vi "Modelo planta H2_V2.vi"() -> ()   [LabVIEW 2024]
uses:
  <vilib>/Platform/TimedLoop/XDataNode/timing_clust.ctl
  <vilib>/Platform/TimedLoop/XDataNode/nitl_modes.ctl
  <vilib>/Platform/TimedLoop/XDataNode/wakeup.ctl
  <vilib>/Modbus/master/Create Master Instance (TCP).vi
  <vilib>/platform/TimedLoop/XDataNode/XDataNode.xnode
  <vilib>/Modbus/master/Modbus Master.lvclass
  <vilib>/OPCUA/NI OPC UA Client.lvlib
  SALICRU_MODBUS.lvlib
  S7-1200_OPCUA.lvlib
  <vilib>/Platform/TimedLoop/XDataNode/XDNodeRunTimeDep.lvlib
  SubVIs/DB_API/DB_API.lvclass
panel:
  out "DB STATUS":bool
  out "Producció d'hidrogen":dbl(graph)
  out "Humedad":dbl format="%#.4g"
  out "Temperatura":dbl format="%#.4g"
  out "Tèrmic\nExtractors":bool
  out "Relé Seguretat":bool
  out "Sobretensions":bool
  out "Baliza verde":bool
  out "Baliza amarilla":bool
  out "Baliza roja":bool
  out "value":cluster{"message":string}
  out "ELYs_Produccio_2":dbl[](array[numeric])
  out "ELYs_Produccio_1":dbl[](array[numeric])
  in  "stop":bool
  out "Corriente S":dbl
  out "Corriente R":dbl
  out "Corriente T":dbl
  out "Salida Vr":dbl
  out "Salida Vt":dbl
  out "Salida Vs":dbl
  out "EV6":bool caption="Not initialized"
  out "EV5":bool caption="Not initialized"
  out "EV4":bool caption="Not initialized"
  out "EV3":bool caption="Idle"
  out "EV2":bool caption="Not initialized"
  out "EV1":bool caption="Stand By"
  out "x-y 4":u32
  out "x-y 3":u32
  in  "Restart INV SALICRU com":bool
  in  "Restart SAI com":bool
  in  "Tab Control":T1(tab)
  out "Prod_elec_total (kg)":dbl format="%#.2g"
  out "E2.1.2":bool caption="Not initialized"
  out "E1.1":bool caption="Maintenance mode"
  out "E2.2.2":bool caption="Not initialized"
  out "E2.3.2":bool caption="Not initialized"
  out "E1.2.2":bool caption="Maintenance mode"
  out "E1.3.2":bool caption="Idle"
  out "Prod_elec_inst (g/s)":dbl format="%#.4g"
  out "Potenica Solar (Display) 2":dbl format="%#.2f"
  out "masa total G Kg 2":dbl format="%#.3f"
  out "P alta 2":dbl format="%.1f"
  out "P baja 2":dbl format="%.1f"
  out "masa total P Kg  2":dbl format="%#.3f"
  in  "SAI":bool caption="Line"
  out "Potenica SAI (Display) 3":dbl format="%#.2f"
  out "Comunicacion SAI":bool
  out "E2.1":bool caption="Not initialized"
  out "E2.2":bool caption="Not initialized"
  out "E1.3":bool caption="Idle"
  out "E1.1,2":bool caption="Maintenance mode"
  out "E2.3":bool caption="Not initialized"
  out "E1.2":bool caption="Maintenance mode"
  out "Energia solar no utilitzada":dbl(graph)
  out "Pressió tanc baixa":dynamicdata(graph)
  out "Potenica Solar (Display)":dbl format="%#.2f"
  out "Producción FC":dbl format="%#_2g"
  out "Prod electrolizadores (display)":dbl format="%#.4g"
  out "P baja":dbl format="%.1f"
  out "masa total G Kg":dbl format="%#.0f"
  out "Potència inversor solar":dynamicdata(graph)
  out "Watimetro ARPA":dbl format="%#.1f"
  out "masa total P Kg":dbl format="%#.1f"
  out "Compresor":bool
  out "P alta":dbl format="%.1f"
  out "H2 generado Total":dbl format="%#.1f"
  out "Producción Solar toral":dbl format="%#.1f"
  out "Energía acum H2 verde":dbl format="%#.1f"
  out "H2 consumido en el lab":dbl=182.6 format="%#.1f"
  out "Energía solar diaría":dbl format="%#.1f"
  out "H2 generado dia":dbl format="%#.1f"
  out "Comunicacion Inversor SALICRU":bool
  out "Tank":dbl(slide) scale=0.0..10.0
  out "CO2":dbl
  out "H2S":dbl
  out "NO2":dbl
  out "O2":dbl
  out "O3":dbl
  out "SO2":dbl
  out "CO":dbl
  out "TVOC":dbl
  out "P tanq alta (barg)":dbl(graph)
  in  "Energía acum H2 verde inicio":dbl=527.0
  in  "Producción Solar total inicio":dbl=3421.0
  in  "H2 generado inicio":dbl=202.8
  out "g H2 consumidos por la FC":dbl
  out "g comprimidos":dbl
  in  "Caudal compresor":dbl
  out "P tanq baja (barg)":dbl(graph)
  in  "Presión ini Tanq baba":dbl=28.0
  in  "Presión ini Tanq alta":dbl=220.0
  out "Energía Solar no usada (kWh)":dbl(graph)
  out "H2 acumulado diario (g)":dbl(graph)
  out "Producción instalan (g/s)":dbl(graph)
  out "Electroli ON":dbl(graph)
  out "Potencia Consumo electroli instan. (kW)":dbl(graph)
  out "Producción diaria (g)":dbl
  out "Producción instalan (g/s)":dbl
  out "Electroli ON":dbl
  out "Potencia Solar Instanta (kW)":dbl(graph)
  # "Seguretat"
  # "EV1"
  # "EV4"
  # "ESTADO ELECTROVÁLVULAS"
  # "EV5"
  # "EV2"
  # "EV3"
  # "EV6"
  # "g"
  # "bar"
  # "bar"
  # "kg"
  # "kWh"
  # "kWh"
  # "Ambiente"
  # "Temperatura"
  # "ºC"
  # "Humedad"
  # "%"
  # "ESTADO ELY"
  # "E1.1"
  # "E2.1"
  # "E1.2"
  # "E2.2"
  # "E2.3"
  # "E1.3"
  # "Modo:"
  # "RESUMEN DE LA PRODUCCIÓN"
  # "Electrolizadores"
  # "Producción\nInstantanea:"
  # "g/s"
  # "Producción\nTotal:"
  # "kg"
  # "SAI PLANTA"
  # "Inversor solar:"
  # "Energía solar:"
  # "kW"
  # "Tanque Alta"
  # "Presión:"
  # "barg"
  # "Kg"
  # "Capacidad:"
  # "Tanque Baja"
  # "Presión:"
  # "barg"
  # "Kg"
  # "Capacidad:"
  # "SAI:"
  # "Potencia (%):"
  # "%"
  # "Hidrògen"
  # "H2 baixa pressió"
  # "H2 alta pressió"
  # "Aigua"
  # "barg"
  # "Tanc baixa pressió"
  # "Tanc alta pressió"
  # "Compressor"
  # "barg"
  # "Solar"
  # "Fuel Cell"
  # "kW"
  # "kW"
  # "kg"
  # "kg"
  # "Electrolizadors"
  # "g/s"
  # "Xarxa electrica"
  # "-"
  # "+"
  # "kW de xarxa"
  # "Producció total d'hidrogen"
  # "Producció d'hidrogen diària"
  # "g"
  # "kg"
  # "Producció total d'energia solar"
  # "Energia solar produïda diària"
  # "kWh"
  # "kWh"
  # "Energia acumulada per H2 verd"
  # "Consum de H2 Lab diari"
  # "g"
  # "kWh"
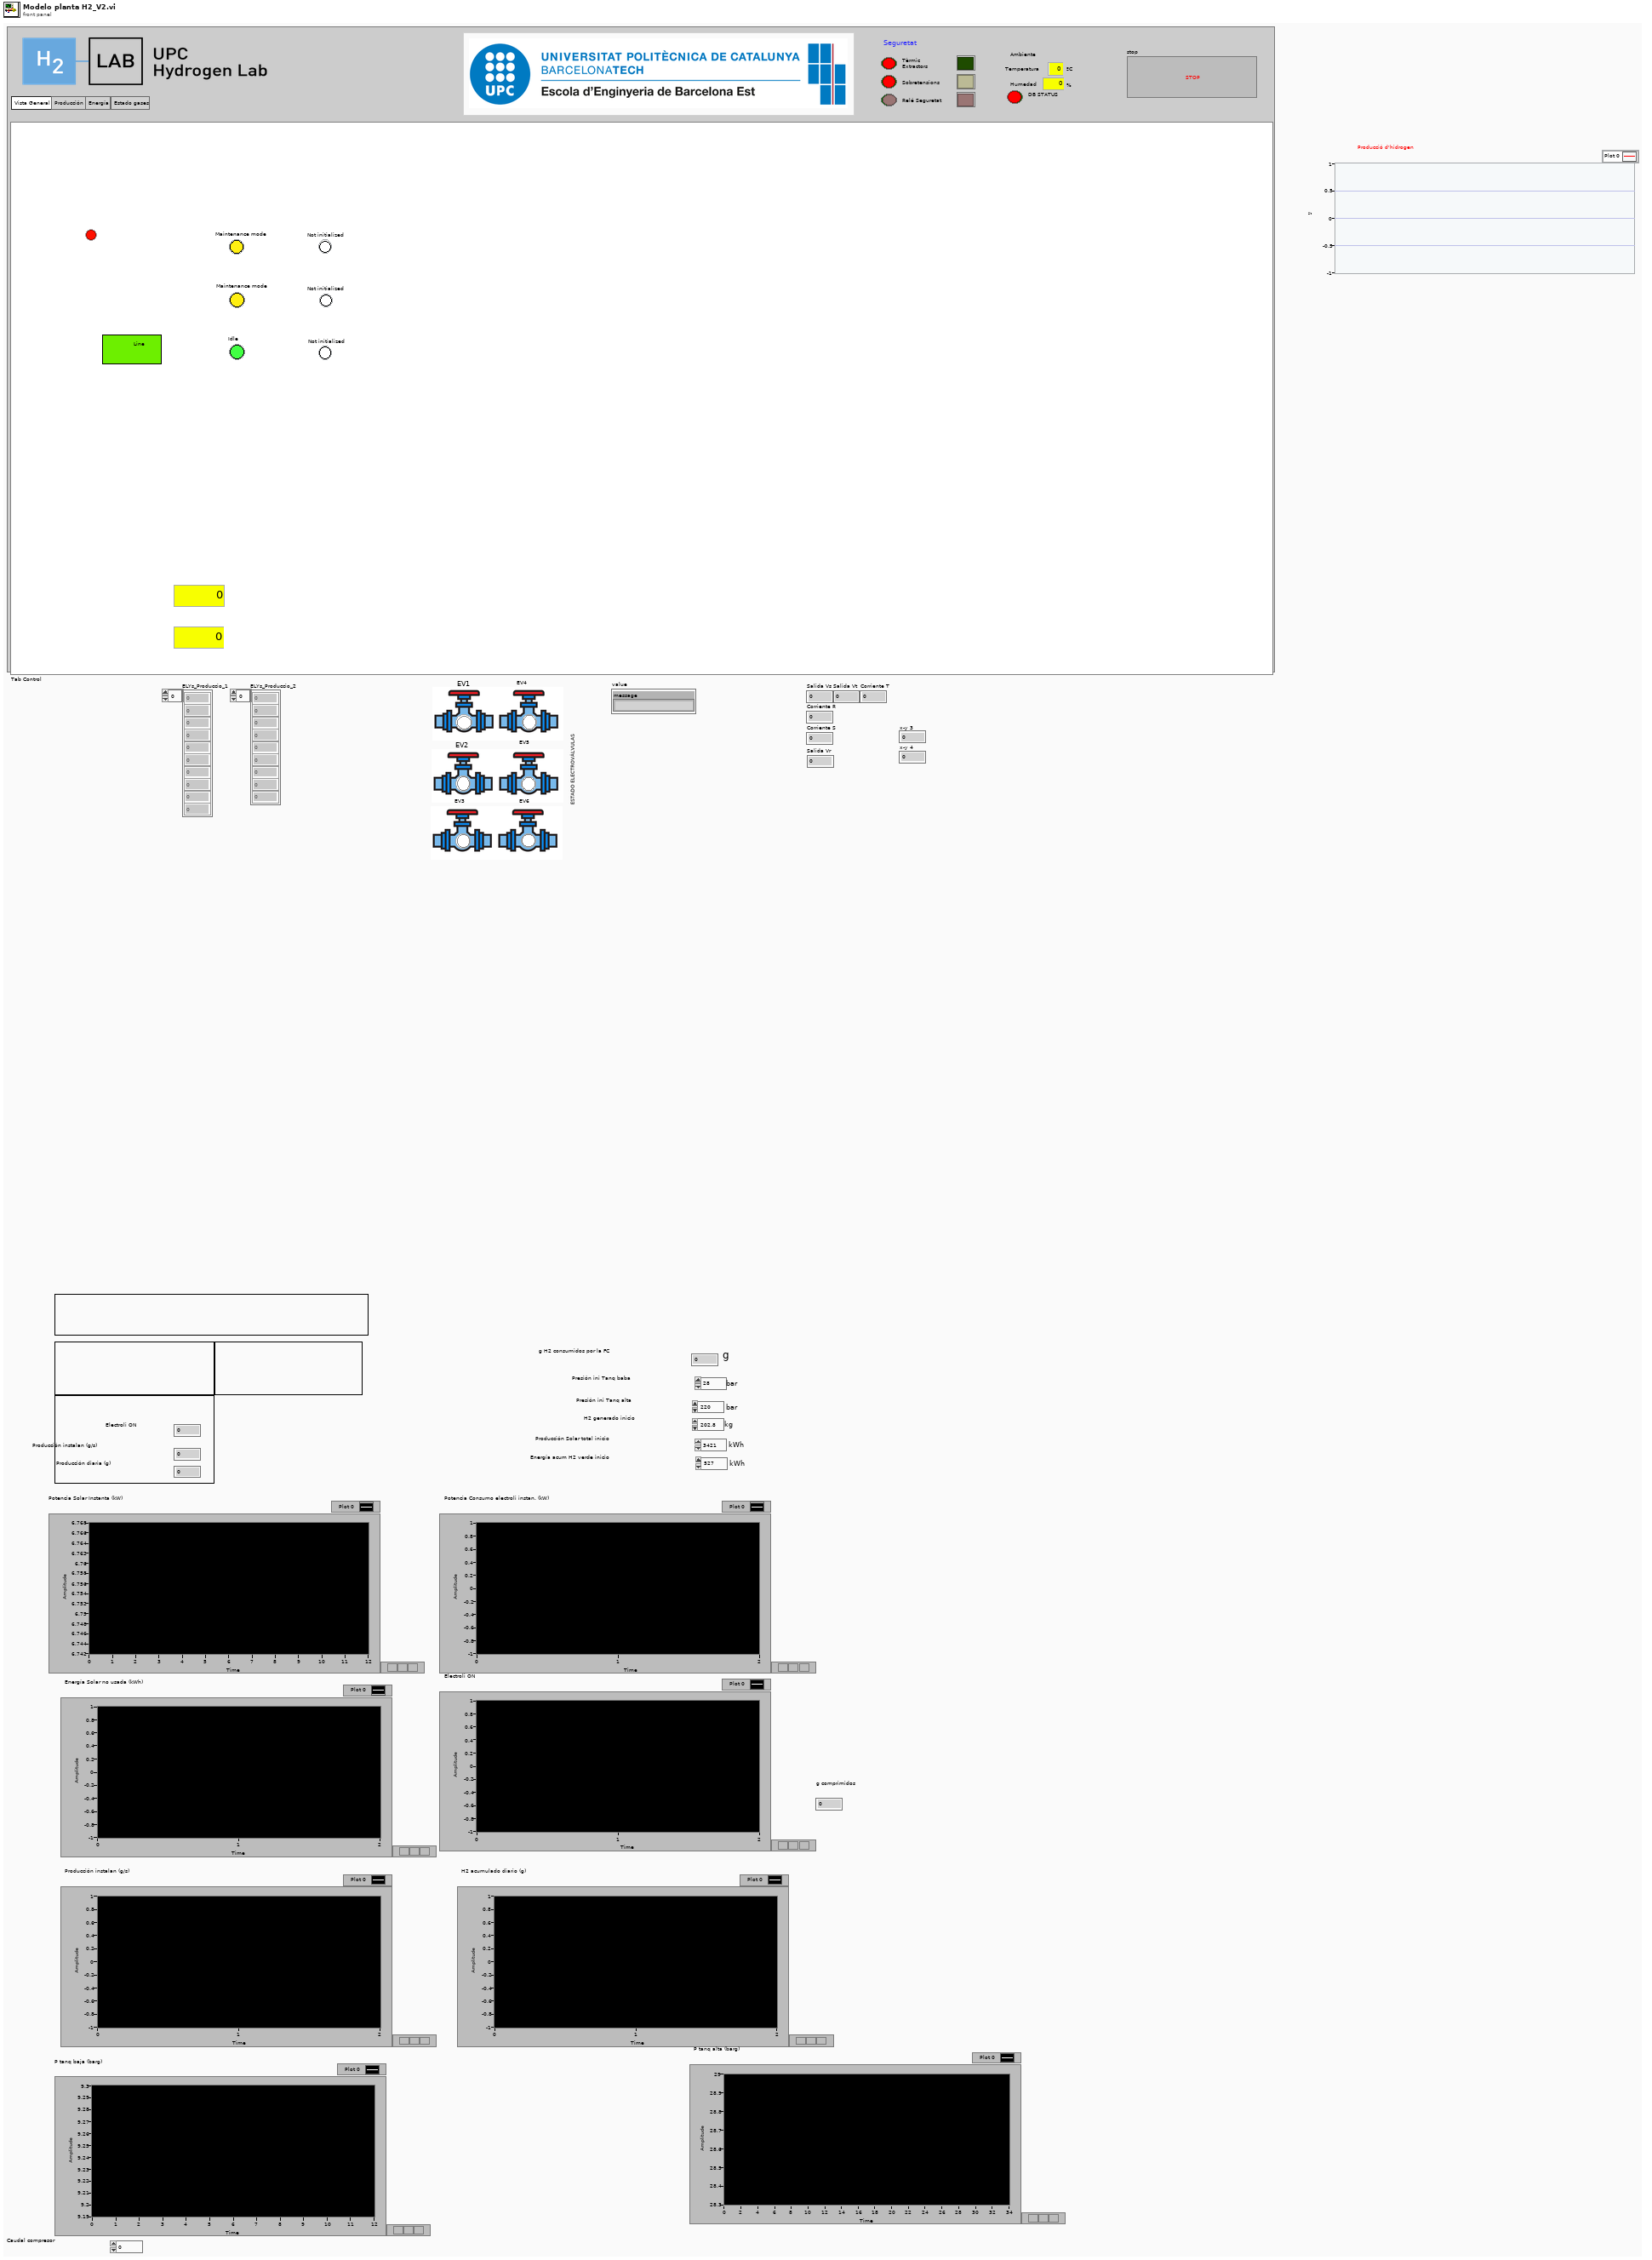
[diagram p1: front panel]
types:
  T1 = enum32{"Vista General", "Producción", "Energía", "Estado gases"}
  T2 = cluster{"message mode":enum16{"None", "Sign", "Sign and Encrypt"}, "security":enum16{"Basic256", "Basic128Rsa15"}}
  T3 = typedef "XDNodeRunTimeDep.lvlib/timing_clust.ctl" = cluster{"Expected End [f-1]":u64, "Actual End [f-1]":u64, "Finished Late? [f-1]":bool, "Expected End [i-1]":u64, "Actual End [i-1]":u64, "Finished Late? [i-1]":bool, "Expected Start [i]":u64, "Actual Start [i]":u64, "Expected Start [f]":u64, "Actual Start [f]":u64, "Source Name":string, "Structure Name":string, "Period":i64, "Deadline":i64, "Offset":i64, "Start":i64, "Priority":i32, "Timeout":i32, "Mode":T4, "Wakeup Reason":T5, "Error":errorcluster, "Source Type":string, "Secondary Source Type":string, "Global End Time":u64, "Global Start Time":u64, "Frame Duration":u64, "Iteration Duration":u64, "Assigned CPU":i32, "I/O Scan Engine Mode":u32}
  T4 = typedef "XDNodeRunTimeDep.lvlib/nitl_modes.ctl" = enum32{"No Change", "Process missed periods, maintain original phase", "Discard missed periods, maintain original phase", "Process missed periods, ignore original phase", "Discard missed periods, ignore original phase"}
  T5 = typedef "XDNodeRunTimeDep.lvlib/wakeup.ctl" = enum32{"Normal", "Aborted", "Asynchronous wakeup", "Timing source error", "Timed loop error", "Timeout"}
  T6 = enum16{"open", "open or create", "create or replace", "create", "open (read-only)"}
  T7 = typedef "OPC UA Client Refnum.ctl" = refnum<k21>
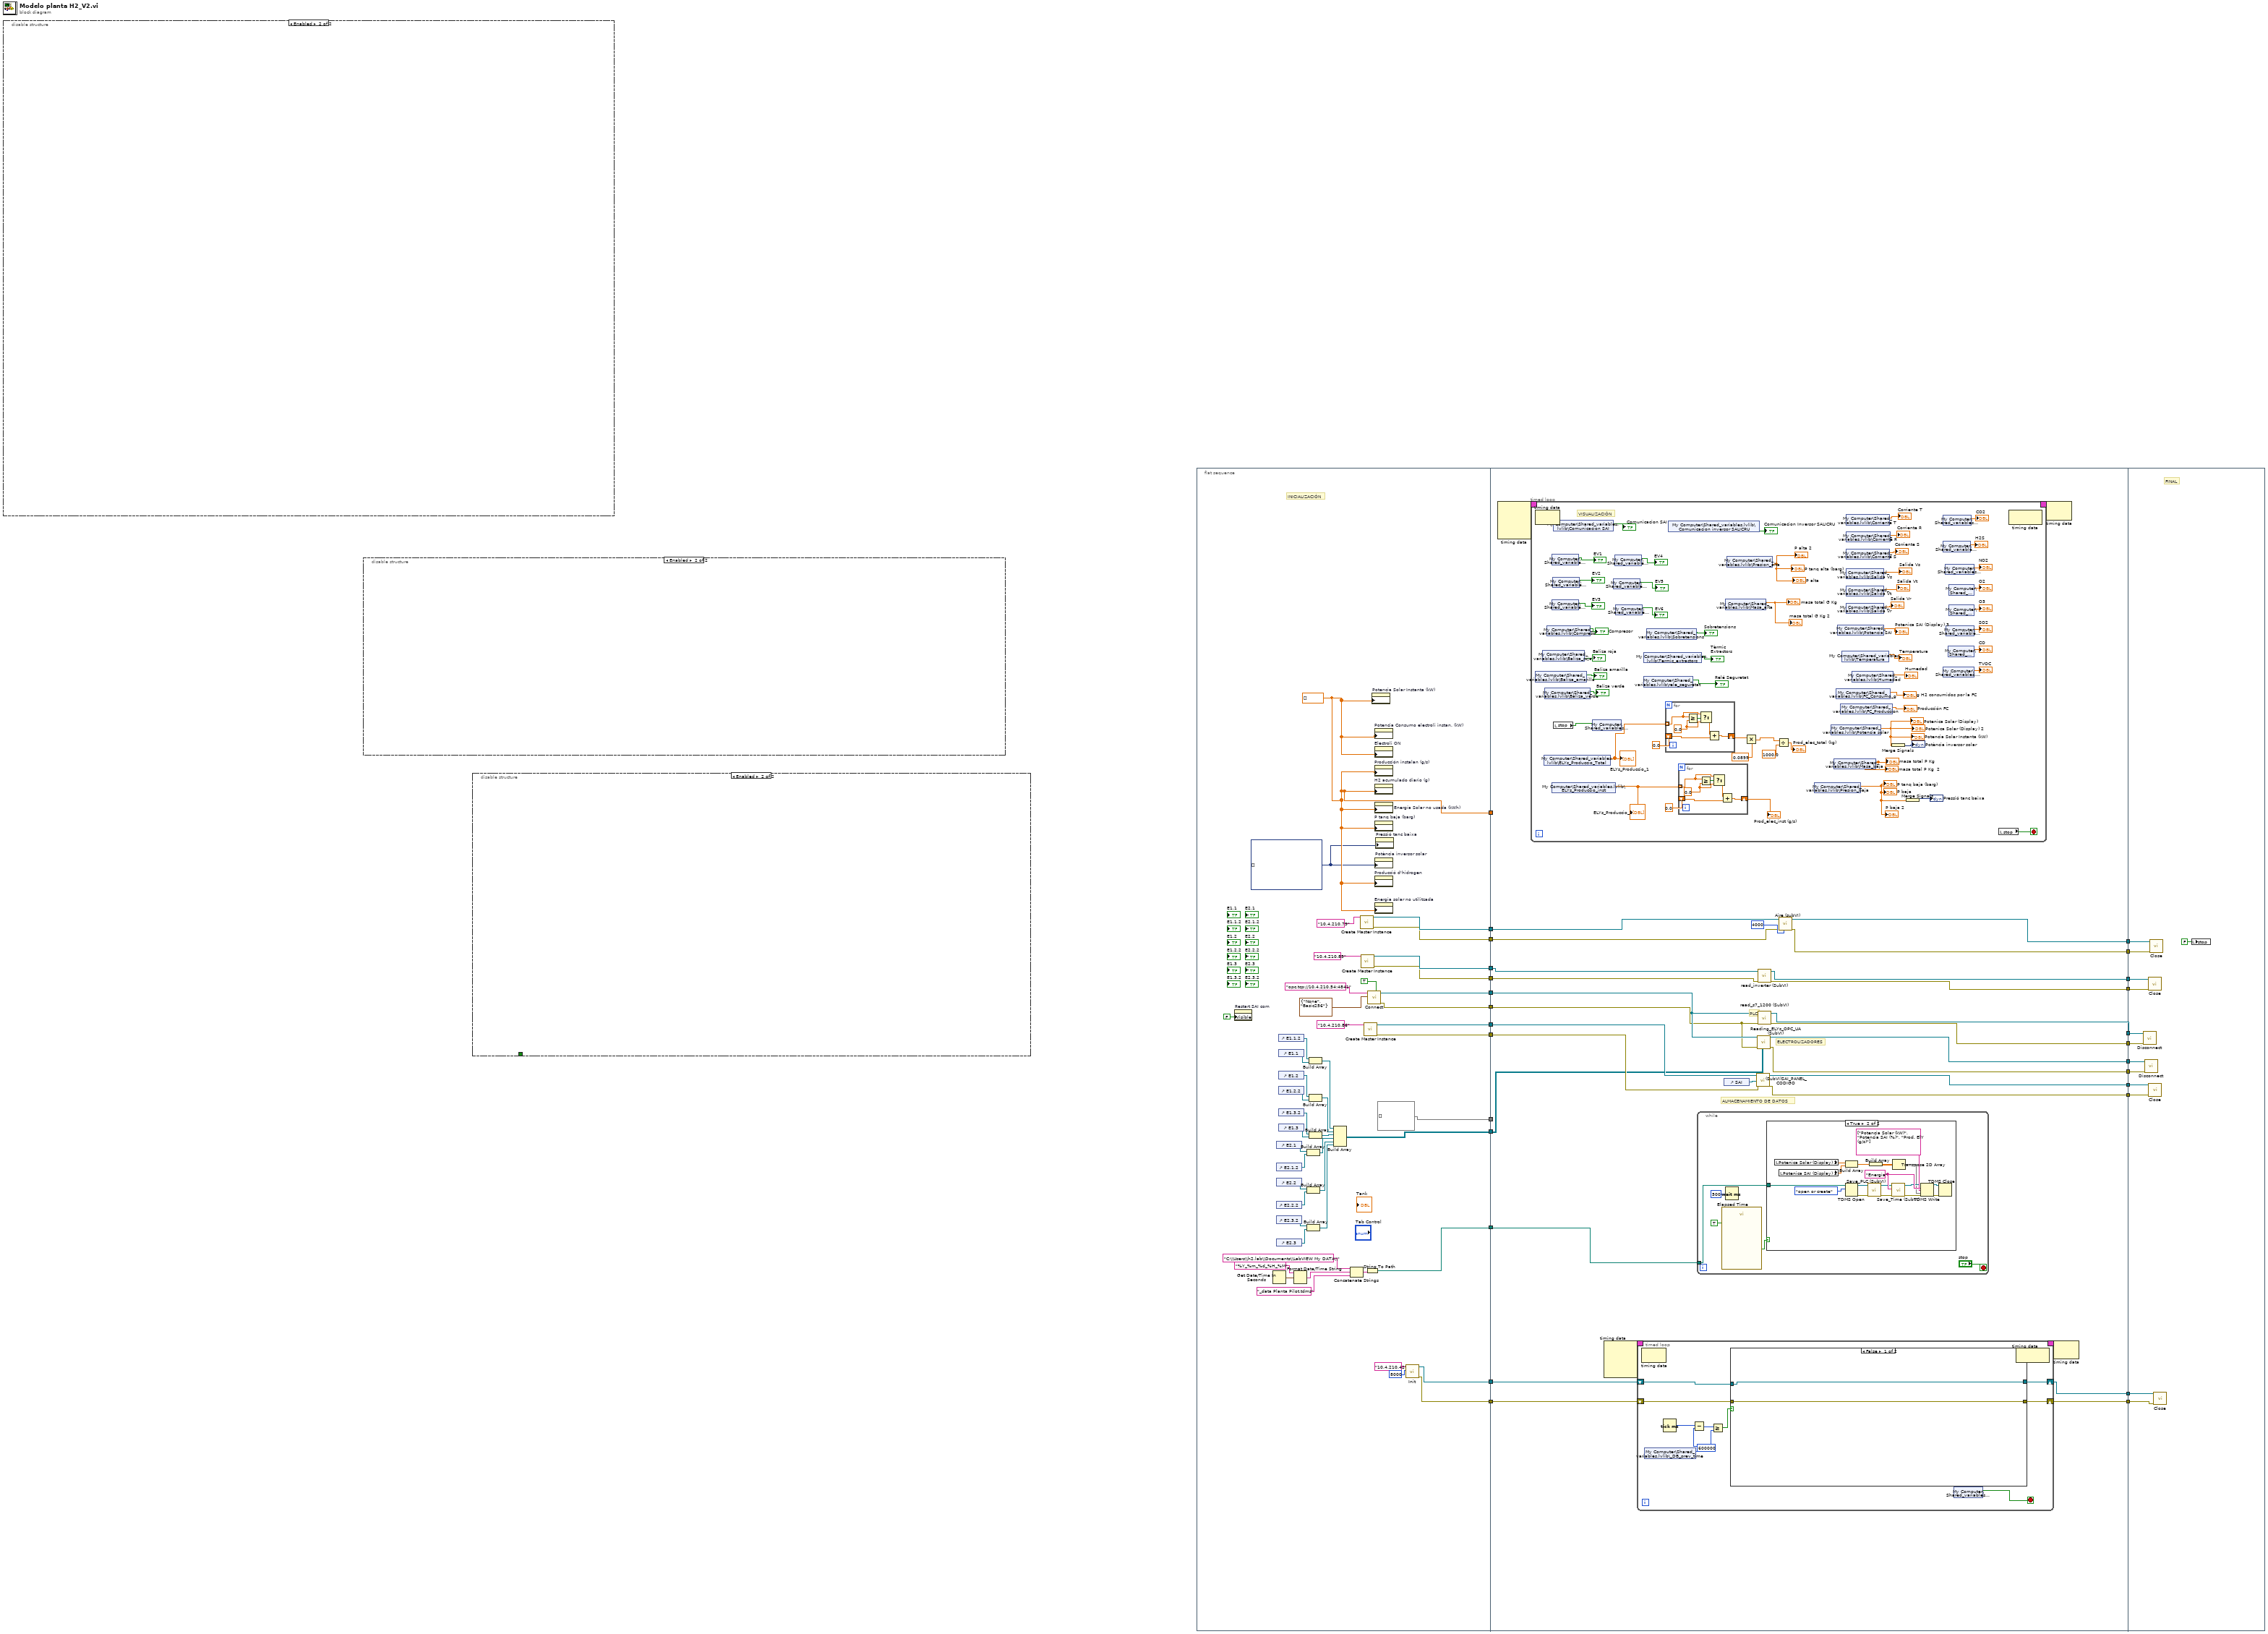
[diagram p0: block diagram]
diagram:
  n1 = disable-structure shown="Enabled" {
    frame Disabled {
      (unwired) 0.95 ("f")
      w43 = 2200.0 ("y")
      # "Totales"
      # "g/s"
      # "2400"
      # "g/s"
      # "Presión tanque de alta"
      # "Presión tanque de baja"
      n2 = local read "Producción diaria (g)"() -> (w38:dbl)
      n3 = local read "Energia solar no utilitzada"() -> (w29:dbl)
      n4 = Random Number (0-1)() -> (number: 0 to 1=w54:dbl)
      n5 = local read "Energía solar diaría"() -> (w33:dbl)
      n6 = Add(x=w54, y=0.0) -> (x+y=w55:dbl)
      n7 = Divide(x=w38, y=1000.0) -> (x/y=w37:dbl)
      n8 = feedback #1(0.0) -> (w101:dbl)
      n9 = Add(x="Caudal compresor", y=w101) -> (x+y=w97:dbl)
      "g comprimidos" <- w97
      n10 = feedback-in #1(w97) -> ()
      n11 = Greater?(x=w55, y=1.0) -> (0:w56:bool)
      n12 = Add(x="H2 generado inicio", y=w37) -> (x+y=→"H2 generado Total":dbl)
      n13 = Add(x="Producción Solar total inicio", y=w33) -> (x+y=→"Producción Solar toral":dbl)
      n14 = Add(x="Energía acum H2 verde inicio", y=w29) -> (x+y=→"Energía acum H2 verde":dbl)
      n15 = Select(t=w55, s=w56, f=0.0) -> (s? t:f=w57:dbl)
      n16 = Divide(x=w97, y=2.0158) -> (x/y=w95:dbl)
      n17 = Compound Arithmetic op=MULTIPLY(w57, 24.0 ("f"), 0.545 ("f"), 0.98 ("f")) -> (w65:dbl)
      n18 = Compound Arithmetic op=MULTIPLY(w95, 0.0831477 ("y"), 293.15 ("y")) -> (w105:dbl)
      n19 = Divide(x=w105, y=810.0) -> (x/y=w104:dbl)
      n20 = Add(x="Presión ini Tanq alta", y=w104) -> (x+y=w99:dbl)
      n21 = Quotient & Remainder(x=w65, y=w43) -> (floor(x/y)=w64:dbl)  [unwired: 1 out]
      n22 = Divide(x=w65, y=1000.0) -> (x/y=w80:dbl)
      n23 = case shown="True" {
        selector: _ -> [_ _]
        tunnel: w64 -> [w109 _]
        tunnel: [w109 _] -> w70
        frame False {
        }
        frame True {
        }
      }
      "Electroli ON" <- w70
      "Electroli ON" <- w70
      n24 = feedback #2(0.0) -> (w79:dbl)
      n25 = Add(x=w80, y=w79) -> (x+y=w78:dbl)
      n26 = feedback-in #2(w78) -> ()
      n27 = Divide(x=w78, y=3600.0) -> (x/y=→"Energía solar diaría":dbl)
      n28 = Multiply(x=w43, y=w70) -> (x*y=w66:dbl)
      n29 = local read "g H2 consumidos por la FC"() -> (w84:dbl)
      n30 = Divide(x=w66, y=1000.0) -> (x/y=w67:dbl)
      "Potencia Consumo electroli instan. (kW)" <- w67
      n31 = Multiply(x=w70, y=0.012486) -> (x*y=w68:dbl)
      "Producción instalan (g/s)" <- w68
      "Producción instalan (g/s)" <- w68
      "Prod electrolizadores (display)" <- w68
      n32 = local read "Producción diaria (g)"() -> (w86:dbl)
      n33 = Subtract(x=w80, y=w67) -> (x-y=w71:dbl)
      n34 = feedback #3(0.0) -> (w61:dbl)
      n35 = Add(x=w68, y=w61) -> (x+y=w82:dbl)
      "Producción diaria (g)" <- w82
      "H2 acumulado diario (g)" <- w82
      "Producció d'hidrogen" <- w82
      "H2 generado dia" <- w82
      n36 = feedback-in #3(w82) -> ()
      n37 = local read "Compresor"() -> (w72:bool)
      n38 = feedback #4(0.0) -> (w62:dbl)
      n39 = Add(x=w71, y=w62) -> (x+y=w63:dbl)
      n40 = feedback-in #4(w63) -> ()
      n41 = Subtract(x=w71, y=0.4) -> (x-y=w74:dbl)
      n42 = Subtract(x=w86, y=w84) -> (x-y=w85:dbl)
      n43 = Subtract(x=w85, y=w97) -> (x-y=w89:dbl)
      n44 = Divide(x=w63, y=3600.0) -> (x/y=→"Energía Solar no usada (kWh)" →"Energia solar no utilitzada":dbl)
      n45 = Divide(x=w89, y=2.0158) -> (x/y=w94:dbl)
      n46 = Select(t=1.5, s=w72, f=0.0 ("t")) -> (s? t:f=w73:dbl)
      n47 = Compound Arithmetic op=MULTIPLY(w94, 0.0831477 ("y"), 293.15 ("y")) -> (w92:dbl)
      n48 = Subtract(x=w74, y=w73) -> (x-y=w75:dbl)
      n49 = Merge Signals() -> ()  [unwired: 1 in, 1 out]
      n50 = Divide(x=w92, y=850.0) -> (x/y=w88:dbl)
      n51 = Add(x=w75, y=0.0) -> (x+y=→"Watimetro ARPA":dbl)
      n52 = Add(x="Presión ini Tanq baba", y=w88) -> (x+y=w83:dbl)
      "H2 consumido en el lab" <- 0.0 ("H2 consumido en el lab")
    }
    frame Enabled {
    }
  }
  n53 = disable-structure shown="Enabled" {
    frame Disabled {
      w111 = FALSE ("Visible")
      w110 = TRUE ("Comunicacion Inversor SALICRU")
      n54 = local write "Restart INV SALICRU com"(w110) -> ()
      n55 = property on="Restart INV SALICRU com" class="Bool (strict)"("Visible"=w111) -> ()  [unwired: 2 in, 2 out]
      n56 = while {
        tunnel: w110 -> [_]
        tunnel: w111 -> [_]
        stop <- w112 stop-if-true
        n57 = Wait (ms)(milliseconds to wait=u32 1000) -> ()  [unwired: 1 out]
        n58 = case shown="True" "Restart INV SALICRU com" {
          frame False {
          }
          frame True {
            n59 = flat-sequence {
              tunnel: [w123] -> w117
              tunnel: [w120] -> w116
              tunnel: [w119] -> w115
              tunnel: w117 -> [w140]
              tunnel: w116 -> [w139]
              tunnel: w115 -> [w138]
              frame #0 {
                w118 = FALSE ("Restart INV SALICRU com")
                # "INVERSOR MODBUS"
                n60 = call-poly <vilib>:"Create Master Instance.vi"("address"="10.4.210.85") -> ("error out"=w121:errorcluster, "TCP master instance"=w122:refnum<class "Modbus Master.lvclass">)  [unwired: 9 in]
                n61 = local write "Restart INV SALICRU com"(w118) -> ()
                n62 = while {
                  shift-right: [w128] -> w120
                  shift-left: w122 -> [w136]
                  shift-right: [w133] -> w123
                  shift-left: w121 -> [w135]
                  tunnel: [w127] -> w119
                  tunnel: w118 -> [_]
                  stop <- w132 stop-if-true
                  # "DELAY BUCLE"
                  n63 = call "read_inverter (SubVI).vi"("error in (no error)"=w135, "Modbus Master in"=w136) -> ("error out"=w133:errorcluster, "Modbus Master out"=w128:refnum<class "Modbus Master.lvclass">)  [unwired: 8 in]
                  n64 = Tick Count (ms)() -> (millisecond timer value=w131:u32)
                  n65 = shared-variable "My Computer\\Shared_variables.lvlib\\Comunicacion inversor SALICRU"() -> (w127:bool)  [unwired: 1 in, 1 out]
                  n66 = Wait (ms)(milliseconds to wait=u32 200) -> ()  [unwired: 1 out]
                  n67 = feedback #5(w131) -> (w130:u32)
                  n68 = feedback-in #5(w131) -> ()
                  n69 = Subtract(x=w131, y=w130) -> (x-y=→"x-y 3":u32)
                  n70 = Not(x=w127) -> (.not. x?=w126:bool)
                  n71 = local read item#-1() -> (w125)
                  n72 = Or(x=w126, y=w125) -> (x .or. y?=w132:bool)
                }
              }
              frame #1 {
                n73 = case shown="True" w138 {
                  tunnel: w140 -> [_ w143]
                  tunnel: w139 -> [_ w142]
                  frame False {
                    n74 = local write "Restart INV SALICRU com"(TRUE ("Restart INV SALICRU com")) -> ()
                  }
                  frame True {
                    n75 = call-dynamic "Close.vi"("error in (no error)"=w143, "Modbus master in"=w142) -> ()  [unwired: 9 in, 1 out]
                  }
                }
                n76 = local write "Comunicacion Inversor SALICRU"(FALSE ("Comunicacion Inversor SALICRU")) -> ()
              }
            }
          }
        }
        n77 = local read item#-1() -> (w112)
      }
    }
    frame Enabled {
    }
  }
  n78 = disable-structure shown="Enabled" {
    disable-tunnel: _ -> [w145 _]
    frame Disabled {
      w144 = TRUE ("Restart SAI com")
      # "SAI SALICRU"
      n79 = local write "Restart SAI com"(w144) -> ()
      n80 = while {
        tunnel: w144 -> [_]
        tunnel: w145 -> [_]
        stop <- w146 stop-if-true
        # "Boton display estado sai"
        n81 = Wait (ms)(milliseconds to wait=u32 1000) -> ()  [unwired: 1 out]
        n82 = case shown="True" "Restart SAI com" {
          frame False {
          }
          frame True {
            n83 = flat-sequence {
              tunnel: [w155] -> w151
              tunnel: [w154] -> w150
              tunnel: [w152] -> w149
              tunnel: w151 -> [w194]
              tunnel: w150 -> [w193]
              tunnel: w149 -> [w191]
              frame #0 {
                w153 = FALSE ("Restart SAI com")
                n84 = call-poly <vilib>:"Create Master Instance.vi"("address"="10.4.210.86") -> ("error out"=w156:errorcluster, "TCP master instance"=w157:refnum<class "Modbus Master.lvclass">)  [unwired: 9 in]
                n85 = while {
                  shift-right: [_] -> w154
                  shift-left: w157 -> [_]
                  shift-right: [_] -> w155
                  shift-left: w156 -> [_]
                  tunnel: w153 -> [_]
                  tunnel: [w160] -> w152
                  stop <- w165 stop-if-true
                  # "DELAY BUCLE"
                  n86 = disable-structure shown="Disabled" {